vi "Data retrieve_plateau_tdms_single.vi"() -> ()   [LabVIEW 2019]
uses:
  <userlib>/LevyLab/LV to ITX/LVtoITX.lvclass
  <userlib>/LevyLab/XY Utilities/xy_utilities.lvlib
  <userlib>/LevyLab/Levylab Instruments/SMOs/Logger.Error/Logger.Error.lvclass
panel:
  in  "index":i32=85
  out "?":dbl[][](graph)
  out "4T conductance single":cluster{dbl[], dbl[]}(graph)
  out "dG4T/dVsg FFT single":cluster{dbl[], "magnitude":dbl[]}(graph)
  out "dG4T/dVsg single":cluster{dbl[], dbl[]}(graph)
  in  "File_index":i32
  in  "index in group":i32
  in  "# per group":i32=1
  in  "Group #":i32=91
  out "V4T":cluster{dbl[], dbl[]}[](graph)
  out "V4T":dbl[][](graph)
  out "dG4T/dVsg":cluster{dbl[], dbl[]}[](graph)
  out "?":dbl[][](graph)
  out "?":dbl[][](graph)
  out "?":dbl[][](graph)
  out "?":dbl[][](graph)
  in  "Vsource":dbl=0.0001
  out "?":dbl[][](graph)
  out "Current":cluster{dbl[], dbl[]}[](graph)
  out "?":dbl[][](graph)
  out "G4T":dbl[][](graph)
  in  "File or Folder Path 2":path=path "C:/Users/muqin/Downloads/0102/05"
  out "4T conductance":cluster{dbl[], dbl[]}[](graph)
  in  "LV to itx":T1={"A"=18, "B"=6, "C"=8, "D"=5, "E"=2, "N1"=3, "N2"=2, "N3"=0, "N4"=0}
  in  "offset":i32
  in  "LV/ITX?":bool=TRUE
  # "FFT part:"
  # "Xaxis"
  # "V4T+"
  # "V4T-"
  # "Drive current"
  # "Vbg/Vsg"
  # "Temp/B"
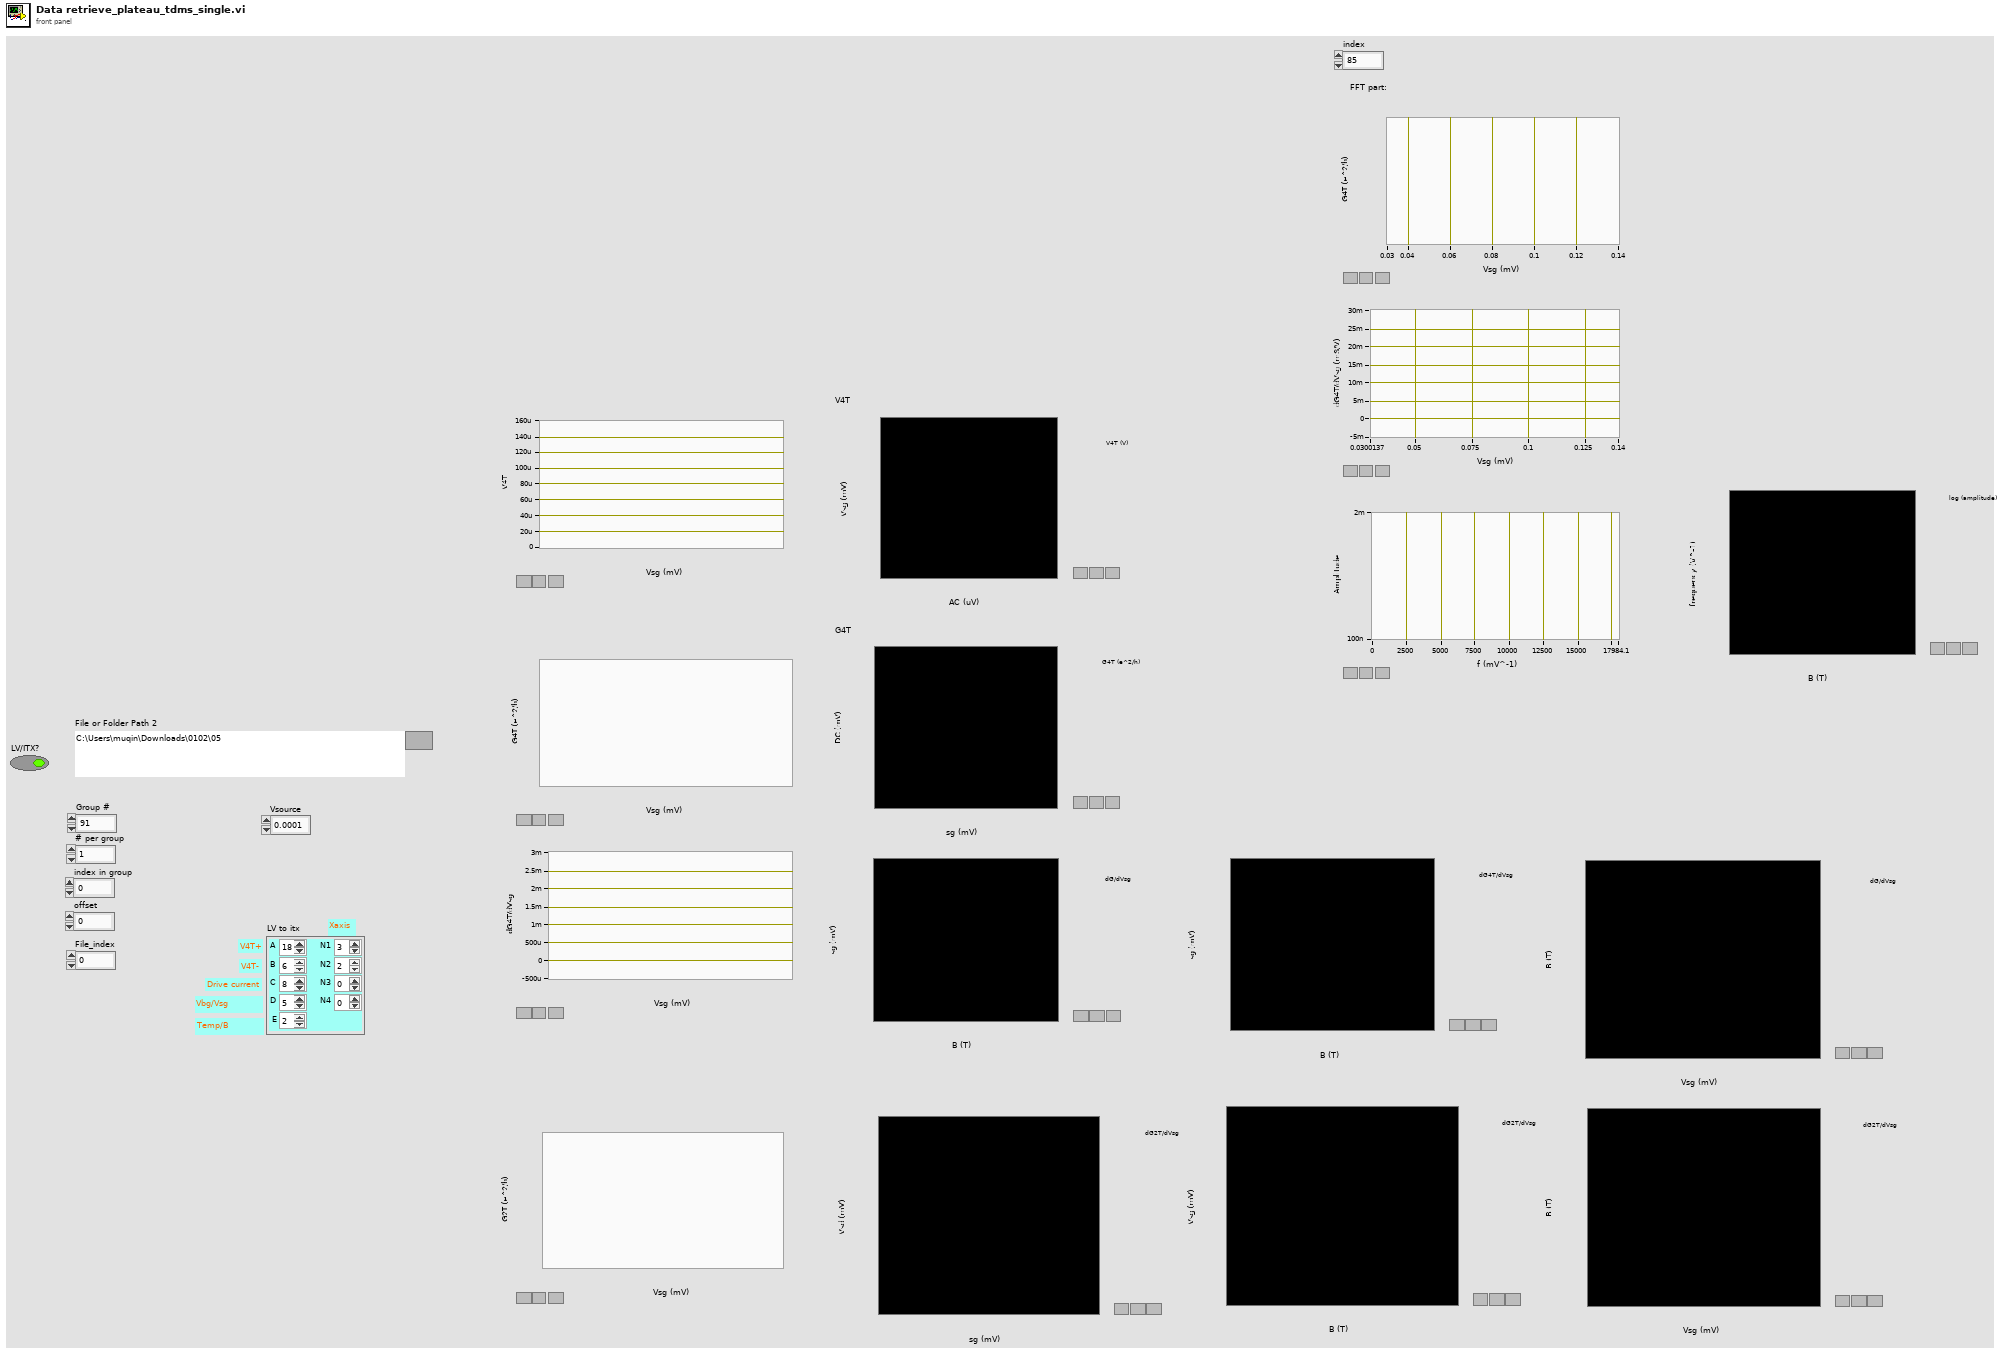
[diagram p1: front panel]
types:
  T1 = cluster{"A":i32, "B":i32, "C":i32, "D":i32, "E":i32, "N1":i32, "N2":i32, "N3":i32, "N4":i32}
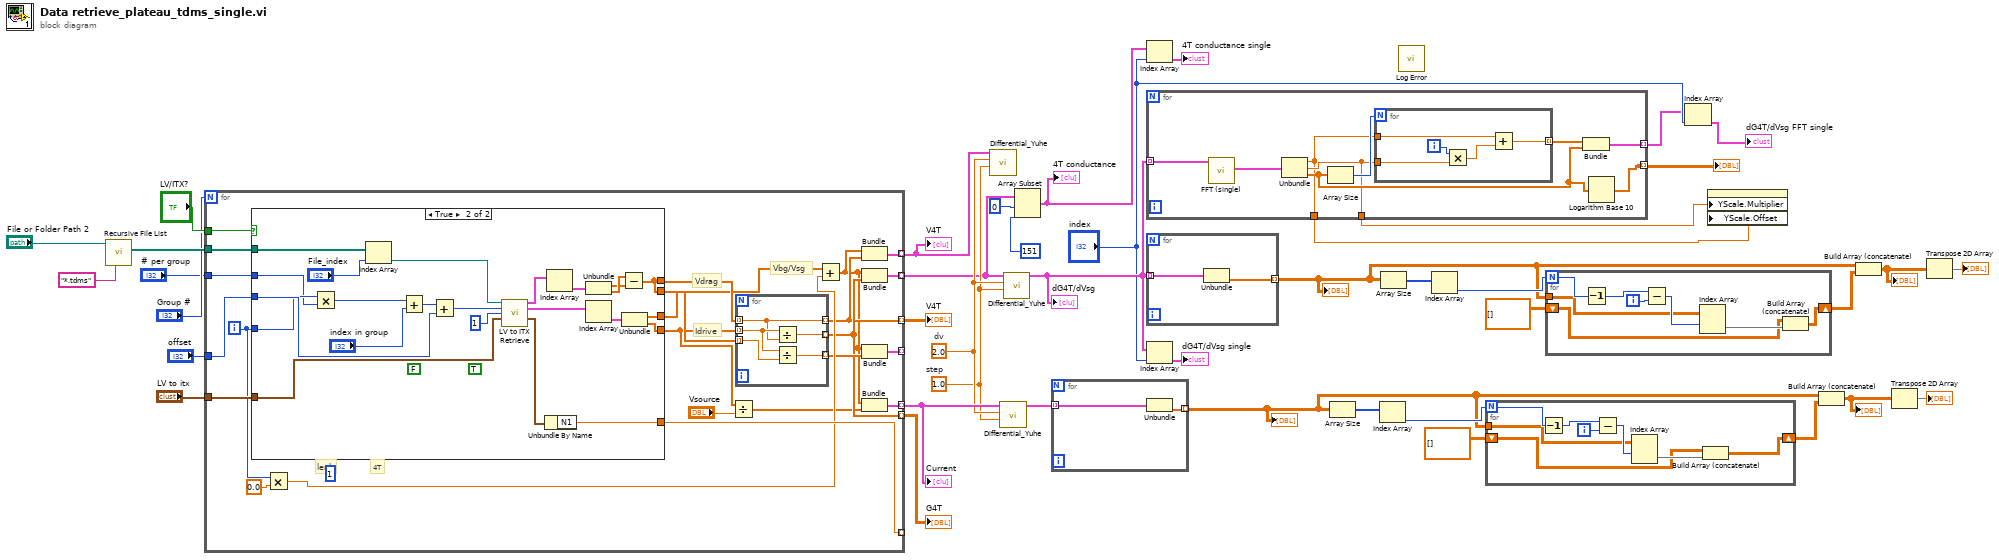
[diagram p0: block diagram]
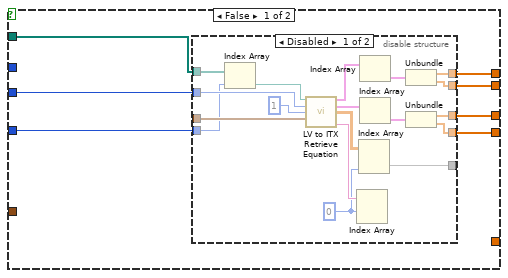
[diagram p2: hidden frame]
diagram:
  w18 = 2.0  # dv
  w17 = 1.0  # step
  n1 = call <vilib>:"Recursive File List.vi"("pattern"="*.tdms", "Folder Path"="File or Folder Path 2") -> ("All Files in Dir"=w39:path[])  [unwired: 5 in, 4 out]
  n2 = for {
    N: "Group #" -> [_]
    tunnel: w39 -> [w65]
    tunnel: "LV to itx" -> [w64]
    tunnel: [w63] -> _ mode=indexing
    tunnel: "offset" -> [w62]
    tunnel: "LV/ITX?" -> [w61]
    tunnel: [w53] -> w13 mode=indexing
    tunnel: [w52] -> _ mode=indexing
    tunnel: [w51] -> w36 mode=indexing
    tunnel: [w50] -> w35 mode=indexing
    tunnel: [w46] -> w21 mode=indexing
    tunnel: [w44] -> w16 mode=indexing
    tunnel: "# per group" -> [w43]
    i -> [w56]
    (unwired) 1 ("disabled index (col)")
    # "Vbg/Vsg"
    # "4T"
    # "leak"
    # "Idrive"
    # "Vdrag"
    n3 = case shown="True" w61 {
      tunnel: w65 -> [w72 w118]
      tunnel: w64 -> [_ w110]
      tunnel: [w75 w104] -> w55
      tunnel: [w74 w105] -> w49
      tunnel: [_ w119] -> w63
      tunnel: [w76 w99] -> w59
      tunnel: [w77 w99] -> w60
      tunnel: w62 -> [w73 w117]
      tunnel: w56 -> [w71 w116]
      tunnel: w43 -> [_ w115]
      frame False {
        n4 = disable-structure shown="Disabled" {
          disable-tunnel: _ -> [w96 _]
          disable-tunnel: [w89 _] -> w77
          disable-tunnel: [w88 _] -> w76
          disable-tunnel: [w87 _] -> w75
          disable-tunnel: [w86 _] -> w74
          disable-tunnel: [w85 _] -> _
          disable-tunnel: w73 -> [w84 _]
          disable-tunnel: w72 -> [w80 _]
          disable-tunnel: w71 -> [w79 _]
          frame Disabled {
            w81 = 0 ("length")
            n5 = Index Array(array=w80, index=w79) -> (element=w78:path)
            n6 = call <userlib>:"LV to ITX  Retrieve Equation.vi"("File or Folder Path"=w78, "offset"=w84, "length"=1, "index"=w96) -> ("y1 vs g"=w94:cluster{dbl[], dbl[]}[], "y2 vs g"=w92:cluster{dbl[], dbl[]}[], "2D"=w90:dbl[][], "Comments"=w83:string)  [unwired: 7 in, 1 out]
            n7 = Index Array(array=w83, index (row)=w81) -> (element=w82)  [unwired: 1 in]
            n8 = Index Array(array=w90, index (col)=w81) -> (element=w85:dbl[])  [unwired: 1 in]
            n9 = Index Array(array=w94) -> (element=w93:cluster{dbl[], dbl[]})  [unwired: 1 in]
            n10 = Index Array(array=w92) -> (element=w91:cluster{dbl[], dbl[]})  [unwired: 1 in]
            n11 = Unbundle(w93) -> (w89:dbl[], w88:dbl[])
            n12 = Unbundle(w91) -> (w87:dbl[], w86:dbl[])
          }
          frame Enabled {
          }
        }
      }
      frame True {
        (unwired) FALSE ("file contains 2D data?")
        (unwired) TRUE ("stop")
        n13 = Multiply(x=w116, y=w115) -> (x*y=w114:i32)
        n14 = Index Array(array=w118, index="File_index") -> (element=w109:path)
        n15 = Add(x=w114, y="index in group") -> (x+y=w112:i32)
        n16 = Add(x=w112, y=w117) -> (x+y=w98:i32)
        n17 = call <userlib>:"LV to ITX  Retrieve.vi"("File or Folder Path"=w109, "offset"=w98, "length"=1, "index"=w110) -> ("A vs B"=w103:cluster{dbl[], dbl[]}[], "C vs D"=w107:cluster{dbl[], dbl[]}[], "N"=w108:cluster{"N1":dbl, "N2":dbl, "N3":dbl, "N4":dbl})  [unwired: 8 in, 1 out]
        n18 = Unbundle By Name(w108) -> ("N1"=w119:dbl)
        n19 = Index Array(array=w103) -> (element=w102:cluster{dbl[], dbl[]})  [unwired: 1 in]
        n20 = Unbundle(w102) -> (w100:dbl[], w101:dbl[])
        n21 = Index Array(array=w107) -> (element=w106:cluster{dbl[], dbl[]})  [unwired: 1 in]
        n22 = Subtract(x=w101, y=w100) -> (x-y=w99:dbl[])
        n23 = Unbundle(w106) -> (w104:dbl[], w105:dbl[])
      }
    }
    n24 = Multiply(x=w56, y=0.0) -> (x*y=w58:dbl)
    n25 = Divide(x=w49, y="Vsource") -> (x/y=w47:dbl[])
    n26 = for {
      tunnel: [w70] -> w51 mode=indexing
      tunnel: [w69] -> w54 mode=indexing
      tunnel: w60 -> [w66] mode=indexing
      tunnel: w59 -> [w68] mode=indexing
      tunnel: w49 -> [w67] mode=indexing
      tunnel: [w66] -> w46 mode=indexing
      n27 = Divide(x=w67, y=w66) -> (x/y=w70:dbl)
      n28 = Divide(x=w67, y=w68) -> (x/y=w69:dbl)
    }
    n29 = Add(x=w55, y=w58) -> (x+y=w45:dbl[])
    n30 = Bundle(w45, w46) -> (w44:cluster{dbl[], dbl[]})  [unwired: 1 in]
    n31 = Bundle(w45, w51) -> (w53:cluster{dbl[], dbl[]})  [unwired: 1 in]
    n32 = Bundle(w45, w54) -> (w52:cluster{dbl[], dbl[]})  [unwired: 1 in]
    n33 = Bundle(w45, w47) -> (w50:cluster{dbl[], dbl[]})  [unwired: 1 in]
  }
  "G4T" <- w36
  "Current" <- w35
  "V4T" <- w21
  "V4T" <- w16
  n34 = call "Differential_Yuhe.vi"("step"=w17, "dv"=w18, "A vs B"=w16) -> ()  [unwired: 8 in, 1 out]
  n35 = call "Differential_Yuhe.vi"("step"=w17, "dv"=w18, "A vs B"=w35) -> ("A vs B 2"=w34:cluster{dbl[], dbl[]}[])  [unwired: 8 in]
  n36 = call "Differential_Yuhe.vi"("step"=w17, "dv"=w18, "A vs B"=w13) -> ("A vs B 2"=w7:cluster{dbl[], dbl[]}[])  [unwired: 8 in]
  "dG4T/dVsg" <- w7
  n37 = Array Subset(array=w13, index=0, length=151) -> (w9:cluster{dbl[], dbl[]}[])
  "4T conductance" <- w9
  n38 = for {
    tunnel: w34 -> [w121] mode=indexing
    tunnel: [w120] -> w22 mode=indexing
    n39 = Unbundle(w121) -> (w120:dbl[])  [unwired: 1 out]
  }
  "?" <- w22
  n40 = Index Array(array=w9, index="index") -> (element=→"4T conductance single":cluster{dbl[], dbl[]})
  n41 = for {
    tunnel: w7 -> [w130] mode=indexing
    tunnel: [w126] -> w2 mode=indexing
    tunnel: [w124] -> w6 mode=indexing
    tunnel: [w123] -> w5
    tunnel: [w122] -> w4
    n42 = call <userlib>:"FFT (single).vi"("XY-data"=w130) -> ("magnitude"=w129:cluster{"f0":dbl, "df":dbl, "magnitude":dbl[]})  [unwired: 7 in, 3 out]
    n43 = Unbundle(w129) -> ("f0"=w122:dbl, "df"=w123:dbl, "magnitude"=w125:dbl[])
    n44 = Array Size(array=w125) -> (size(s)=w127:i32)
    n45 = for {
      N: w127 -> [_]
      tunnel: w123 -> [w135]
      tunnel: [w131] -> w128 mode=indexing
      tunnel: w122 -> [w133]
      i -> [w134]
      n46 = Multiply(x=w134, y=w135) -> (x*y=w132:dbl)
      n47 = Add(x=w133, y=w132) -> (x+y=w131:dbl)
    }
    n48 = Bundle(w128, "magnitude"=w125) -> (w126:cluster{dbl[], "magnitude":dbl[]})  [unwired: 1 in]
    n49 = Logarithm Base 10(1:w125) -> (0:w124:dbl[])
  }
  "?" <- w6
  n50 = for {
    tunnel: w7 -> [w137] mode=indexing
    tunnel: [w136] -> w14 mode=indexing
    n51 = Unbundle(w137) -> (w136:dbl[])  [unwired: 1 out]
  }
  "?" <- w14
  n52 = Index Array(array=w7, index="index") -> (element=→"dG4T/dVsg single":cluster{dbl[], dbl[]})
  n53 = Array Size(array=w22) -> (size(s)=w29:i32[])
  n54 = Index Array(array=w29) -> (element=w28:i32)  [unwired: 1 in]
  n55 = Array Size(array=w14) -> (size(s)=w32:i32[])
  n56 = call <userlib>:"Log Error.vi"() -> ()  [unwired: 10 in, 2 out]
  n57 = Index Array(array=w32) -> (element=w31:i32)  [unwired: 1 in]
  n58 = for {
    N: w28 -> [w145]
    tunnel: w22 -> [w141]
    shift-right: [w139] -> w23
    shift-left: dbl[][] [] -> [w138]
    i -> [w142]
    n59 = Decrement(x=w145) -> (x-1=w143:i32)
    n60 = Subtract(x=w143, y=w142) -> (x-y=w144:i32)
    n61 = Index Array(array=w141, index (row)=w144) -> (element=w140:dbl[])  [unwired: 1 in]
    n62 = Build Array (concatenate)(w138, w140) -> (w139:dbl[][])
  }
  n63 = for {
    N: w31 -> [w153]
    tunnel: w14 -> [w149]
    shift-right: [w147] -> w15
    shift-left: dbl[][] [] -> [w146]
    i -> [w150]
    n64 = Decrement(x=w153) -> (x-1=w151:i32)
    n65 = Subtract(x=w151, y=w150) -> (x-y=w152:i32)
    n66 = Index Array(array=w149, index (row)=w152) -> (element=w148:dbl[])  [unwired: 1 in]
    n67 = Build Array (concatenate)(w146, w148) -> (w147:dbl[][])
  }
  n68 = Index Array(array=w2, index="index") -> (element=→"dG4T/dVsg FFT single":cluster{dbl[], "magnitude":dbl[]})
  n69 = property class="IntGraph (strict)"("YScale.Multiplier"=w5, "YScale.Offset"=w4) -> ()  [unwired: 2 in, 2 out]
  n70 = Build Array (concatenate)(w22, w23) -> (w25:dbl[][])
  "?" <- w25
  n71 = Build Array (concatenate)(w14, w15) -> (w27:dbl[][])
  "?" <- w27
  n72 = Transpose 2D Array(2D array=w25) -> (transposed array=→"?":dbl[][])
  n73 = Transpose 2D Array(2D array=w27) -> (transposed array=→"?":dbl[][])
